vi "UHR-Fleezers Control (host) - Avogadro v2.vi"() -> ()   [LabVIEW 2014] (continued)
        n2315 = local read "Setpoints (V)"() -> (w3599:cluster{"Set 1":dbl, "Set 2":dbl})
        n2316 = Unbundle By Name(w3584) -> ("kappa_x (pN/nm)"=w3595:dbl, "kappa_y (pN/nm)"=w3594:dbl)
        n2317 = Unbundle By Name(w3591) -> ("kappa_x (pN/nm)"=w3593:dbl, "kappa_y (pN/nm)"=w3592:dbl)
        n2318 = Unbundle By Name(w3599) -> ("Set 1"=w3602:dbl, "Set 2"=w3601:dbl)
        n2319 = case shown="True" "Scale intensities" {
          tunnel: w3602 -> [w3616 w3629]
          tunnel: w3601 -> [w3615 w3622]
          tunnel: "Scaling factor" -> [w3612 w3617]
          tunnel: [w3614 w3628] -> w3597
          tunnel: [w3613 w3627] -> w3596
          tunnel: w3595 -> [w3611 w3623]
          tunnel: w3594 -> [w3610 w3624]
          tunnel: w3593 -> [w3609 w3625]
          tunnel: w3592 -> [w3608 w3626]
          tunnel: [w3607 w3621] -> w3590
          tunnel: [w3606 w3620] -> w3589
          tunnel: [w3605 w3619] -> w3588
          tunnel: [w3604 w3618] -> w3587
          frame False {
            n2320 = Divide(x=w3616, y=w3612) -> (x/y=w3614:dbl)
            n2321 = Divide(x=w3608, y=w3612) -> (x/y=w3604:dbl)
            n2322 = Divide(x=w3615, y=w3612) -> (x/y=w3613:dbl)
            n2323 = Divide(x=w3611, y=w3612) -> (x/y=w3607:dbl)
            n2324 = Divide(x=w3610, y=w3612) -> (x/y=w3606:dbl)
            n2325 = Divide(x=w3609, y=w3612) -> (x/y=w3605:dbl)
          }
          frame True {
            n2326 = Multiply(x=w3629, y=w3617) -> (x*y=w3628:dbl)
            n2327 = Multiply(x=w3622, y=w3617) -> (x*y=w3627:dbl)
            n2328 = Multiply(x=w3626, y=w3617) -> (x*y=w3618:dbl)
            n2329 = Multiply(x=w3623, y=w3617) -> (x*y=w3621:dbl)
            n2330 = Multiply(x=w3624, y=w3617) -> (x*y=w3620:dbl)
            n2331 = Multiply(x=w3625, y=w3617) -> (x*y=w3619:dbl)
          }
        }
        n2332 = Bundle By Name(cluster=w3584, "kappa_x (pN/nm)"=w3590, "kappa_y (pN/nm)"=w3589) -> (w3586:T12)
        n2333 = Bundle By Name(cluster=w3591, "kappa_x (pN/nm)"=w3588, "kappa_y (pN/nm)"=w3587) -> (w3585:T12)
        n2334 = Bundle By Name(cluster=w3599, "Set 1"=w3597, "Set 2"=w3596) -> (w3598:cluster{"Set 1":dbl, "Set 2":dbl})
        n2335 = property on="T1 calibration" class="Clust (strict)"("Val(Sgnl)"=w3586) -> ()  [unwired: 2 in, 2 out]
        n2336 = property on="T2 calibration" class="Clust (strict)"("Val(Sgnl)"=w3585) -> ()  [unwired: 2 in, 2 out]
        n2337 = property on="Setpoints (V)" class="Clust (strict)"("Val(Sgnl)"=w3598) -> ()  [unwired: 2 in, 2 out]
      }
      event "Piezo X at\n Scan position (V)": Value Change {
        n2338 = event-data() -> ()  [unwired: 7 out]
        n2339 = local read "AOM position for scan (MHz)"() -> (w3638:dbl)
        n2340 = local read "Piezo Trap X cal (nm/V)"() -> (w3632:dbl)
        n2341 = local read "AOM X Cal (nm/MHz)"() -> (w3635:dbl)
        n2342 = Subtract(x=w3638, y=60.0) -> (x-y=w3636:dbl)
        n2343 = Multiply(x=w3636, y=w3635) -> (x*y=w3633:dbl)
        n2344 = Multiply(x="Piezo X at\n Scan position (V)", y=w3632) -> (x*y=w3634:dbl)
        n2345 = Subtract(x=w3634, y=w3633) -> (x-y=w3631:dbl)
        n2346 = Divide(x=w3631, y=w3632) -> (x/y=→"Piezo trap x\noffset (V)":dbl)
      }
      event "Shift offset": Value Change {
        # "This events shifts the offset values by the currently measured values. For a quick way of correcting for changes in offsets"
        n2347 = event-data() -> ()  [unwired: 7 out]
        n2348 = local read "Multi-MCL offset array"() -> (w3661:T30)
        n2349 = local read "Offset file step size"() -> (w3649:dbl)
        n2350 = local read "MCL offset scanning range (V)"() -> (w3650:T4)
        n2351 = local write "Shift offset"(FALSE) -> ()
        n2352 = local read "Trap position array"() -> (w3662:dbl[])
        n2353 = Build Array(1, 0, 4, 3, 11, 10) -> (w3653:i32[])
        n2354 = local read "Values"() -> (w3654:dbl[])
        n2355 = for {
          tunnel: w3654 -> [w3666]
          tunnel: w3653 -> [w3665] mode=indexing
          tunnel: [w3664] -> w3652 mode=indexing
          n2356 = Index Array(array=w3666, index=w3665) -> (element=w3664:dbl)
        }
        n2357 = call "select offset array.vi"("MCL offset scanning range (V)"=w3650, "Offset File step size"=w3649, "Multi-MCL offset array"=w3661, "Trap position array"=w3662) -> ("Out offsets"=w3651:dbl[])  [unwired: 1 out]
        n2358 = Subtract(x=w3652, y=w3651) -> (x-y=w3641:dbl[])
        n2359 = local read "Raw offsets"() -> (w3648:dbl[])
        n2360 = Negate(x=w3641) -> (-x=w3640:dbl[])
        n2361 = call "generate multiple MCL offset.vi"("Offset array"=w3648, "offset file step size"=w3649, "MCL offset scanning range (V)"=w3650, "Corrections"=w3640) -> ("B_X mean out"=w3642:dbl[], "A_X mean out"=w3643:dbl[], "Output array"=w3647:T30)
        n2362 = local write "Multi-MCL offset array"(w3647) -> ()
        n2363 = local read "B factor"() -> (w3644:dbl)
        n2364 = Multiply(x=w3642, y=w3644) -> (x*y=w3646:dbl[])
        n2365 = Subtract(x=w3643, y=w3646) -> (x-y=w3645:dbl[])
        n2366 = property on="Setpoint offset\ncorrection values" class="Arr (strict)"("Val(Sgnl)"=w3645) -> ()  [unwired: 2 in, 2 out]
      }
    }
    "error out 2" <- w1816
    n2367 = node-c288() -> ()  [unwired: 2 out]
  }
  n2368 = node-c288() -> (w64:T42)  [unwired: 4 out]
  n2369 = timed-loop "Mouse control: trap position (AOM deflection), set confocal spot from image" {
    tunnel: [w3667] -> w69
    timing: w64 -> [_]
    timing-out: [_] -> w63
    tunnel: w26 -> [w3668]
    stop <- w3667 stop-if-true
    n2370 = node-c288() -> ()  [unwired: 2 out]
    n2371 = event shown="[0] \"Pane\": Mouse Down" {
      selector: _ -> [_ _ _ _]
      dyn-events: _ -> [_ _ _ _]
      timeout: _ -> [_ _ _ _]
      tunnel: w3668 -> [w3671 _ _ _]
      tunnel: [_ _ TRUE _] -> w3667
      event Mouse Down {
        n2372 = event-data() -> ("Time"=w3673:u32, "Coords"=w3672:T16, "Button"=w3674:u16)  [unwired: 6 out]
        n2373 = case shown="1" w3674 {
          tunnel: w3673 -> [_ _ w3799]
          tunnel: w3672 -> [_ w3711 w3797]
          tunnel: w3671 -> [_ _ w3793]
          frame 0, Default {
          }
          frame 1 {
            n2374 = property on="APD 2" class="ImageControl"() -> ("Displayed Image Position"=w3681:cluster{"Left":i32, "Top":i32})  [unwired: 2 in, 2 out]
            n2375 = property on="APD 1" class="ImageControl"() -> ("Displayed Image Position"=w3710:cluster{"Left":i32, "Top":i32})  [unwired: 2 in, 2 out]
            n2376 = property on="Detection Laser X" class="ImageControl"() -> ("Displayed Image Position"=w3707:cluster{"Left":i32, "Top":i32})  [unwired: 2 in, 2 out]
            n2377 = property on="Detection Laser Y" class="ImageControl"() -> ("Displayed Image Position"=w3706:cluster{"Left":i32, "Top":i32})  [unwired: 2 in, 2 out]
            n2378 = property on="APD 2" class="ImageControl"() -> ("Displayed Image Size"=w3680:cluster{"Width":u32, "Height":u32})  [unwired: 2 in, 2 out]
            n2379 = property on="APD 1" class="ImageControl"() -> ("Displayed Image Size"=w3708:cluster{"Width":u32, "Height":u32})  [unwired: 2 in, 2 out]
            n2380 = property on="Detection Laser X" class="ImageControl"() -> ("Displayed Image Size"=w3709:cluster{"Width":u32, "Height":u32})  [unwired: 2 in, 2 out]
            n2381 = property on="Detection Laser Y" class="ImageControl"() -> ("Displayed Image Size"=w3705:cluster{"Width":u32, "Height":u32})  [unwired: 2 in, 2 out]
            n2382 = Unbundle By Name(w3680) -> ("Width"=w3677:u32, "Height"=w3676:u32)
            n2383 = Unbundle By Name(w3681) -> ("Left"=w3679:i32, "Top"=w3678:i32)
            n2384 = Unbundle By Name(w3708) -> ("Width"=w3702:u32, "Height"=w3701:u32)
            n2385 = Unbundle By Name(w3709) -> ("Width"=w3698:u32, "Height"=w3697:u32)
            n2386 = Unbundle By Name(w3705) -> ("Width"=w3694:u32, "Height"=w3693:u32)
            n2387 = Unbundle By Name(w3710) -> ("Left"=w3704:i32, "Top"=w3703:i32)
            n2388 = Unbundle By Name(w3707) -> ("Left"=w3700:i32, "Top"=w3699:i32)
            n2389 = Unbundle By Name(w3706) -> ("Left"=w3696:i32, "Top"=w3695:i32)
            n2390 = Bundle("Left"=w3679, "Top"=w3678, "Width"=w3677, "Height"=w3676) -> (w3675:T58)  [unwired: 1 in]
            n2391 = Bundle("Left"=w3704, "Top"=w3703, "Width"=w3702, "Height"=w3701) -> (w3692:T58)  [unwired: 1 in]
            n2392 = Bundle("Left"=w3700, "Top"=w3699, "Width"=w3698, "Height"=w3697) -> (w3691:T58)  [unwired: 1 in]
            n2393 = Bundle("Left"=w3696, "Top"=w3695, "Width"=w3694, "Height"=w3693) -> (w3690:T58)  [unwired: 1 in]
            n2394 = Build Cluster Array(w3675, w3692, w3691, w3690) -> (w3689:T59)
            n2395 = for {
              tunnel: w3711 -> [w3722]
              tunnel: w3689 -> [w3723] mode=indexing
              shift-right: [w3720] -> w3687
              shift-left: TRUE -> [w3721]
              shift-right: [w3719] -> w3685
              shift-left: _ -> [w3715]
              shift-right: [w3718] -> w3684
              shift-left: _ -> [w3714]
              shift-right: [w3717] -> w3683
              shift-left: _ -> [w3713]
              shift-right: [w3716] -> w3682
              shift-left: _ -> [w3712]
              n2396 = case shown="True" w3721 {
                selector: w3721 -> [w3728 _]
                tunnel: w3723 -> [_ w3737]
                tunnel: w3722 -> [_ w3735]
                tunnel: [w3728 w3733] -> w3720
                tunnel: [w3727 w3732] -> w3719
                tunnel: [w3726 w3731] -> w3718
                tunnel: [w3725 w3730] -> w3717
                tunnel: [w3724 w3729] -> w3716
                tunnel: w3715 -> [w3727 _]
                tunnel: w3714 -> [w3726 _]
                tunnel: w3713 -> [w3725 _]
                tunnel: w3712 -> [w3724 _]
                frame False {
                }
                frame True {
                  n2397 = Unbundle(w3737) -> (w3736:T58)
                  n2398 = call "isclickinwindow.vi"("Image Param"=w3736, "Point32"=w3735) -> ("4 Y"=w3729:i32, "3 Height"=w3730:i32, "2 X"=w3731:i32, "1 Width"=w3732:i32, "In image?"=w3734:bool)  [unwired: 1 in]
                  n2399 = Not(x=w3734) -> (.not. x?=w3733:bool)
                }
              }
            }
            n2400 = Not(x=w3687) -> (.not. x?=w3686:bool)
            n2401 = case shown="True" w3686 {
              tunnel: w3684 -> [_ w3755]
              tunnel: w3682 -> [_ w3754]
              tunnel: w3685 -> [_ w3753]
              tunnel: w3683 -> [_ w3752]
              frame False {
              }
              frame True {
                w3742 = FALSE ("Get Point")
                n2402 = local read "Scan steps (MCL)"() -> (w3738:u64)
                n2403 = local read "Actual MCL Inc (V)"() -> (w3751:dbl)
                n2404 = local read "Scan lines (y)"() -> (w3756:u64)
                n2405 = Divide "Y Pix/step"(x=w3752, y=w3756) -> (x/y=w3762:dbl)
                n2406 = Divide "X pix/step"(x=w3753, y=w3738) -> (x/y=w3760:dbl)
                n2407 = Divide "Y V/pix"(x=w3751, y=w3762) -> (x/y=w3761:dbl)
                n2408 = local read "Initial Y"() -> (w3769:dbl)
                n2409 = Divide "Y half step offset"(x=w3751, y=2.0) -> (x/y=w3740:dbl)
                n2410 = Divide "X half step offset"(x=w3751, y=2.0) -> (x/y=w3758:dbl)
                n2411 = Divide "X V/pix"(x=w3751, y=w3760) -> (x/y=w3759:dbl)
                n2412 = Multiply(x=w3754, y=w3761) -> (x*y=w3770:dbl)
                n2413 = Negate(x=w3740) -> (-x=w3763:dbl)
                n2414 = Multiply(x=w3751, y=w3738) -> (x*y=w3765:dbl)
                n2415 = Multiply(x=w3759, y=w3755) -> (x*y=w3767:dbl)
                n2416 = Negate(x=w3758) -> (-x=w3757:dbl)
                n2417 = Compound Arithmetic op=ADD(w3763, w3770, w3769) -> (w3743:dbl)
                "Pointer Y (V)" <- w3743
                n2418 = local read "Initial X"() -> (w3768:dbl)
                n2419 = Negate(x=w3767) -> (-x=w3766:dbl)
                n2420 = Compound Arithmetic op=ADD(w3757, w3765, w3768, w3766) -> (w3744:dbl)
                "Pointer X (V)" <- w3744
                n2421 = case shown="True" "Set High F Confocal Spot (X-Y)" {
                  tunnel: w3744 -> [_ w3791]
                  tunnel: w3743 -> [_ w3792]
                  frame False {
                  }
                  frame True {
                    "Confocal Y 2 (V)" <- w3792
                    "Confocal X 2 (V)" <- w3791
                  }
                }
                n2422 = local read "Scan trap 3 or Fl?"() -> (w3741:bool)
                n2423 = Or(x="Set X Only", y="Set Confocal Spot (X-Y)") -> (x .or. y?=w3747:bool)
                n2424 = Or(x="Set Confocal Spot (X-Y)", y="Set Y Only") -> (x .or. y?=w3746:bool)
                n2425 = case shown="False" w3741 {
                  tunnel: w3747 -> [w3774 w3780]
                  tunnel: w3746 -> [w3773 w3779]
                  tunnel: w3744 -> [w3772 w3777]
                  tunnel: w3743 -> [w3771 w3778]
                  frame False {
                    n2426 = case shown="True" w3773 {
                      tunnel: w3771 -> [_ w3776]
                      frame False {
                      }
                      frame True {
                        n2427 = property on="AO1" class="Slide (strict)"("Val(Sgnl)"=w3776) -> ()  [unwired: 2 in, 2 out]
                        "Confocal Y 1 (V)" <- w3776
                      }
                    }
                    n2428 = case shown="True" w3774 {
                      tunnel: w3772 -> [_ w3775]
                      frame False {
                      }
                      frame True {
                        n2429 = property on="AO2" class="Slide (strict)"("Val(Sgnl)"=w3775) -> ()  [unwired: 2 in, 2 out]
                        "Confocal X 1 (V)" <- w3775
                      }
                    }
                  }
                  frame True {
                    n2430 = case shown="True" w3779 {
                      tunnel: w3778 -> [_ w3781]
                      frame False {
                      }
                      frame True {
                        n2431 = property on="Piezo trap y\noffset (V)" class="DigNum (strict)"("Val(Sgnl)"=w3781) -> ()  [unwired: 2 in, 2 out]
                      }
                    }
                    n2432 = case shown="True" w3780 {
                      tunnel: w3777 -> [_ w3786]
                      frame False {
                      }
                      frame True {
                        n2433 = local read "AOM X Cal (nm/MHz)"() -> (w3787:dbl)
                        n2434 = local read "Trap Delta (MHz)"() -> (w3789:dbl)
                        n2435 = Subtract(x=30.0, y=w3789) -> (x-y=w3788:dbl)
                        n2436 = Multiply(x=w3788, y=w3787) -> (x*y=w3784:dbl)
                        n2437 = local read "Piezo Trap X cal (nm/V)"() -> (w3783:dbl)
                        n2438 = Divide(x=w3784, y=w3783) -> (x/y=w3782:dbl)
                        n2439 = Subtract(x=w3786, y=w3782) -> (x-y=w3785:dbl)
                        n2440 = property on="Piezo trap x\noffset (V)" class="DigNum (strict)"("Val(Sgnl)"=w3785) -> ()  [unwired: 2 in, 2 out]
                      }
                    }
                  }
                }
                n2441 = local write "Set High F Confocal Spot (X-Y)"(w3742) -> ()
                n2442 = local write "Set Confocal Spot (X-Y)"(w3742) -> ()
                n2443 = local write "Set X Only"(w3742) -> ()
                n2444 = local write "Set Y Only"(w3742) -> ()
              }
            }
          }
          frame 3 {
            n2445 = local read "BD 2 Frequency 1 (MHz)"() -> (w3794:dbl)
            n2446 = local read "BD 1 Frequency 1 (MHz)"() -> (w3795:dbl)
            n2447 = local write "Manipulating Trap"(TRUE ("Manipulating Trap")) -> ()
            n2448 = local write "Coords"(T16 {"Horizontal"=0, "Vertical"=0} ("Coords")) -> ()
            n2449 = while {
              tunnel: w3799 -> [w3804]
              tunnel: w3797 -> [w3803]
              tunnel: w3795 -> [w3802]
              tunnel: w3794 -> [w3801]
              tunnel: w3793 -> [w3800]
              stop <- w3805 stop-if-true
              n2450 = event shown="[0] \"Pane\": Mouse Move" {
                selector: _ -> [_ _]
                dyn-events: _ -> [_ _]
                timeout: _ -> [_ _]
                tunnel: ["Force Manip Abort" w3869] -> w3805
                tunnel: w3804 -> [w3812 _]
                tunnel: w3803 -> [w3810 _]
                tunnel: w3802 -> [w3809 _]
                tunnel: w3801 -> [w3808 _]
                tunnel: w3800 -> [w3806 _]
                event Mouse Move {
                  n2451 = event-data() -> ("Time"=w3813:u32, "Coords"=w3814:T16)  [unwired: 3 out]
                  n2452 = Less?(x=w3813, y=w3812) -> (x < y?=w3811:bool)
                  n2453 = case "Makes sure old motion events prior to mouse click aren't used" shown="False" w3811 {
                    tunnel: w3814 -> [w3856 _]
                    tunnel: w3810 -> [w3857 _]
                    tunnel: w3809 -> [w3831 _]
                    tunnel: w3808 -> [w3830 _]
                    tunnel: w3806 -> [w3815 _]
                    frame False {
                      n2454 = Subtract(x=w3856, y=w3857) -> (x-y=w3855:T16)
                      "Coords" <- w3855
                      n2455 = local read "Y RF Frequency Limits (MHz)"() -> (w3816:T26)
                      n2456 = To Double Precision Float(number=w3855) -> (double precision float=w3854:cluster{"Horizontal":dbl, "Vertical":dbl})
                      n2457 = Multiply(x=cluster{"Horizontal":dbl, "Vertical":dbl} {"Horizontal"=-1.0, "Vertical"=1.0}, y="Manipulation Scaling") -> (x*y=w3850:cluster{"Horizontal":dbl, "Vertical":dbl})
                      n2458 = local read "X RF Frequency Limits (MHz)"() -> (w3817:T26)
                      n2459 = Multiply(x=w3854, y=w3850) -> (x*y=w3852:cluster{"Horizontal":dbl, "Vertical":dbl})
                      n2460 = Unbundle By Name(w3852) -> ("Horizontal"=w3847:dbl, "Vertical"=w3851:dbl)
                      n2461 = Unbundle By Name(w3816) -> ("Maximum"=w3819:dbl, "Minimum"=w3818:dbl)
                      n2462 = Boolean To (0,1)(Boolean="Manip. X?") -> (0, 1=w3845:i16)
                      n2463 = Boolean To (0,1)(Boolean="Manip. Y?") -> (0, 1=w3842:i16)
                      n2464 = local read "BD 1 Frequency 2 (MHz)"() -> (w3833:dbl)
                      n2465 = Multiply(x=w3851, y=w3842) -> (x*y=w3844:dbl)
                      n2466 = Multiply(x=w3845, y=w3847) -> (x*y=w3848:dbl)
                      n2467 = local read "BD 2 Frequency 2 (MHz)"() -> (w3832:dbl)
                      n2468 = Unbundle By Name(w3817) -> ("Maximum"=w3821:dbl, "Minimum"=w3820:dbl)
                      n2469 = Add(x=w3830, y=w3844) -> (x+y=w3823:dbl)
                      n2470 = Add(x=w3831, y=w3848) -> (x+y=w3825:dbl)
                      n2471 = In Range and Coerce(upper limit=w3821, x=w3825, lower limit=w3820) -> (coerced(x)=w3824:dbl)  [unwired: 1 out]
                      n2472 = In Range and Coerce(upper limit=w3819, x=w3823, lower limit=w3818) -> (coerced(x)=w3822:dbl)  [unwired: 1 out]
                      n2473 = Subtract(x=w3824, y=w3833) -> (x-y=w3841:dbl)
                      n2474 = Subtract(x=w3822, y=w3832) -> (x-y=w3840:dbl)
                      n2475 = Square(x=w3841) -> (x^2=w3839:dbl)
                      n2476 = Square(x=w3840) -> (x^2=w3838:dbl)
                      n2477 = Add(x=w3839, y=w3838) -> (x+y=w3837:dbl)
                      n2478 = Square Root(x=w3837) -> (sqrt(x)=w3834:dbl)
                      n2479 = In Range and Coerce(upper limit="Limit Max (MHz)", x=w3834, lower limit="Limit Min (MHz)") -> (In Range?=w3827:bool)  [unwired: 1 out]
                      n2480 = Not(x="Limits Enable") -> (.not. x?=w3826:bool)
                      n2481 = Or(x=w3827, y=w3826) -> (x .or. y?=w3828:bool)
                      n2482 = case shown="True" w3828 {
                        tunnel: w3834 -> [_ w3859]
                        tunnel: w3824 -> [_ w3866]
                        tunnel: w3833 -> [_ w3865]
                        tunnel: w3822 -> [_ w3864]
                        tunnel: w3832 -> [_ w3863]
                        tunnel: w3817 -> [_ w3861]
                        tunnel: w3816 -> [_ w3860]
                        tunnel: w3815 -> [_ w3858]
                        frame False {
                        }
                        frame True {
                          n2483 = local read "BD 1 Frequency 3 (MHz)"() -> (w3867:dbl)
                          n2484 = local read "BD 2 Frequency 3 (MHz)"() -> (w3862:dbl)
                          n2485 = local write "Trap Delta (MHz)"(w3859) -> ()
                          n2486 = call "set RF board frequency - interlace.vi"("Board 2 Frequency Limits"=w3860, "Board 1 Frequency Limits"=w3861, "FPGA VI Reference In"=w3858, "Board 2 Frequency 3 (MHz)"=w3862, "Board 1 Frequency 3 (MHz)"=w3867, "Board 2 Frequency 2 (MHz)"=w3863, "Board 2 Frequency 1 (MHz)"=w3864, "Board 1 Frequency 2 (MHz)"=w3865, "Board 1 Frequency 1  (MHz)"=w3866) -> ()  [unwired: 1 in, 2 out]
                          n2487 = local write "BD 2 Frequency 1 (MHz)"(w3864) -> ()
                          n2488 = local write "BD 1 Frequency 1 (MHz)"(w3866) -> ()
                        }
                      }
                    }
                    frame True {
                    }
                  }
                }
                event Mouse Up {
                  n2489 = event-data() -> ("Button"=w3868:u16)  [unwired: 8 out]
                  n2490 = case shown="3" w3868 {
                    tunnel: [FALSE TRUE] -> w3869
                    frame 0, Default {
                    }
                    frame 3 {
                      n2491 = local read "Trap Delta (MHz)"() -> (w3871:dbl)
                      n2492 = property on="Initial delta (MHz)" class="DigNum (strict)"("Val(Sgnl)"=w3871) -> ()  [unwired: 2 in, 2 out]
                      n2493 = local write "Manipulating Trap"(FALSE ("Manipulating Trap")) -> ()
                    }
                  }
                }
              }
            }
          }
        }
      }
      event Timeout {
        n2494 = event-data() -> ()  [unwired: 4 out]
      }
      event "Stop All": Mouse Down {
        n2495 = event-data() -> ()  [unwired: 9 out]
      }
      event Mouse Move {
        n2496 = event-data() -> ()  [unwired: 6 out]
      }
    }
    n2497 = node-c288() -> ()  [unwired: 2 out]
  }
  n2498 = node-c288(i64 1 ("Period"), 1 ("Processor")) -> (w68:T42)  [unwired: 2 in, 2 out]
  n2499 = node-c288(3 ("Processor")) -> (w60:T42)  [unwired: 3 out]
  n2500 = timed-loop "Oscillate Trap/AOM (fishing, conjugate plane alignment)" {
    tunnel: [w3877] -> w65
    timing: w60 -> [_]
    timing-out: [_] -> w59
    tunnel: w26 -> [w3876]
    tunnel: w3 -> [w3875]
    stop <- w3877 stop-if-true
    n2501 = node-c288() -> ()  [unwired: 2 out]
    n2502 = event shown="[2] \"Start assembly line\": Value Change" {
      selector: _ -> [_ _ _ _]
      dyn-events: _ -> [_ _ _ _]
      timeout: _ -> [_ _ _ _]
      tunnel: [FALSE ("Stop All") _ _ w4550] -> w3877
      tunnel: w3876 -> [w3880 _ _ _]
      tunnel: w3875 -> [_ _ w4485 _]
      event "Oscillate Set 1", "Fish for Tether": Value Change {
        n2503 = event-data() -> ()  [unwired: 6 out]
        n2504 = local read "Oscillate Set 1"() -> (w3884:bool)
        n2505 = Or(x=w3884, y="Fish for Tether") -> (x .or. y?=w3882:bool)
        n2506 = case shown="True" w3882 {
          tunnel: "Fish for Tether" -> [_ w3887]
          tunnel: w3880 -> [_ w3885]
          frame False {
          }
          frame True {
            n2507 = case shown="True" w3887 {
              selector: w3887 -> [w3890 w3896]
              tunnel: [w3890 w3896] -> w3886
              frame False {
              }
              frame True {
                n2508 = local write "Scan axis 2"(TRUE) -> ()
                n2509 = local write "Tether"(FALSE ("Tether")) -> ()
                n2510 = local read "Flow ON during cal?"() -> (w3891:bool)
                n2511 = property on="Trap Delta (MHz)" class="DigNum (strict)"("Val(Sgnl)"="Furthest Delta (MHz)") -> ()  [unwired: 2 in, 2 out]
                n2512 = Or(x="Flow ON during \nfishing?", y=w3891) -> (x .or. y?=w3892:bool)
                n2513 = Wait (ms)(milliseconds to wait=u32 500) -> ()  [unwired: 1 out]
                n2514 = property on="Sample Channel\nFlow" class="Bool (strict)"("Val(Sgnl)"=w3892) -> ()  [unwired: 2 in, 2 out]
              }
            }
            n2515 = node-c288() -> (w3889:T42)  [unwired: 1 in, 3 out]
            n2516 = timed-loop "Oscillate AOD" {
              timing: w3889 -> [_]
              timing-out: [_] -> w3888
              tunnel: w3886 -> [w3900]
              tunnel: w3885 -> [w3899]
              i -> [w3908]
              stop <- w3906 stop-if-true
              n2517 = node-c288() -> (w3907:i64)  [unwired: 1 out]
              n2518 = flat-sequence {
                tunnel: w3908 -> [w3935]
                tunnel: w3907 -> [w3934]
                tunnel: w3900 -> [w3918]
                tunnel: [w3918] -> w3905
                tunnel: [w3917] -> w3904
                tunnel: [w3916] -> w3903
                tunnel: [w3913] -> w3901
                tunnel: w3899 -> [w3909]
                tunnel: w3905 -> [w3982]
                tunnel: w3904 -> [w3980]
                tunnel: w3903 -> [w3979]
                tunnel: [w3978] -> w3902
                tunnel: w3901 -> [w3977]
                tunnel: [w4054] -> w3906
                tunnel: w3902 -> [w4053]
                frame #0 {
                  # "w (rad/s)"
                  # "t (s)"
                  n2519 = Divide(x=w3934, y=i64 1000) -> (x/y=w3910:dbl)
                  n2520 = local read "BD 1 Frequency 2 (MHz)"() -> (w3912:dbl)
                  n2521 = Multiply(x="Osc. freq. (Hz)", y=6.283185307179586) -> (x*y=w3932:dbl)
                  n2522 = Multiply(x=w3910, y=w3935) -> (x*y=w3931:dbl)
                  n2523 = Multiply(x=w3932, y=w3931) -> (x*y=w3915:dbl)
                  n2524 = local read "BD 1 Frequency 1 (MHz)"() -> (w3920:dbl)
                  n2525 = case shown="True" w3918 {
                    tunnel: w3915 -> [w3941 w3960]
                    tunnel: w3920 -> [_ w3968]
                    tunnel: w3912 -> [_ w3969]
                    tunnel: [w3938 w3964] -> w3911
                    tunnel: [FALSE w3942] -> w3916
                    tunnel: [0.0 w3956] -> w3913
                    frame False {
                      n2526 = Sine(x=w3941) -> (sin(x)=w3939:dbl)
                      n2527 = Multiply(x=w3939, y="Osc. amp. (MHz)") -> (x*y=w3938:dbl)
                    }
                    frame True {
                      # "trap position goes from 0 to 1 (0 is when it is furthest away, 1 is when closest)\nso we want to test for tether only when farther away, or x < 1"
                      # "quit if taking too long"
                      # "oscillate the trap"
                      # "Test for tether"
                      n2528 = local read "Vec Mean of T1 T2"() -> (w3945:dbl[])
                      "Trigger Signal" <- w3945
                      n2529 = Cosine(x=w3960) -> (cos(x)=w3972:dbl)
                      n2530 = Subtract(x=w3969, y=w3968) -> (x-y=w3967:dbl)
                      n2531 = Decrement(x=w3972) -> (x-1=w3971:dbl)
                      n2532 = Subtract(x=w3967, y="Closest Delta (MHz)") -> (x-y=w3965:dbl)
                      n2533 = Divide(x=w3971, y=-2.0) -> (x/y=w3955:dbl)
                      n2534 = Greater?(x=w3945, y="Stop F (pN)") -> (0:w3962:bool[])
                      n2535 = Multiply(x=w3955, y=w3965) -> (x*y=w3964:dbl)
                      n2536 = Less?(x=w3955, y="Fish mask thresh") -> (x < y?=w3954:bool)
                      n2537 = Boolean To (0,1)(Boolean=w3954) -> (0, 1=w3952:i16)
                      n2538 = Multiply(x=w3952, y=w3945) -> (x*y=w3951:dbl[])
                      n2539 = Divide(x=w3960, y=6.283185307179586) -> (x/y=w3959:dbl)
                      n2540 = Round Toward +Infinity(x=w3959) -> (ceil(x): smallest int >= x=w3956:dbl)
                      "Attempts" <- w3956
                      n2541 = Greater?(x=w3951, y="Stop F (pN) (mask)") -> (0:w3949:bool[])
                      n2542 = Or Array Elements(Boolean array=w3962) -> (logical OR=w3947:bool)
                      n2543 = Or Array Elements(Boolean array=w3949) -> (logical OR=w3946:bool)
                      n2544 = Greater?(x=w3956, y="Attempt Limit") -> (0:w3958:bool)
                      n2545 = case shown="True" w3958 {
                        frame False {
                        }
                        frame True {
                          n2546 = local write "Fish for Tether"(FALSE ("Fish for Tether")) -> ()
                          n2547 = call <vilib>:"Beep.vi"() -> ()  [unwired: 3 in, 9 out]
                          n2548 = local read "Messages"() -> (w3974:string)
                          n2549 = call "Update messages.vi"("Message to add"="Tether fishing timeout." ("Messages"), "Old message string"=w3974) -> ("New message string"=→"Messages":string)
                        }
                      }
                      n2550 = Select(t=w3947, s="Normal (on) or masked test (off)", f=w3946) -> (s? t:f=w3944:bool)
                      n2551 = And(x="Stop Fishing When Tether", y=w3944) -> (x .and. y?=w3942:bool)
                    }
                  }
                  n2552 = local read "BD 2 Frequency 1 (MHz)"() -> (w3919:dbl)
                  n2553 = Select(t=w3920, s="Scan axis 2", f=w3919) -> (s? t:f=w3923:dbl)
                  n2554 = Add(x=w3911, y=w3923) -> (x+y=w3917:dbl)
                  n2555 = Select(t=w3917, s="Scan axis 2", f=w3920) -> (s? t:f=w3926:dbl)
                  n2556 = Select(t=w3919, s="Scan axis 2", f=w3917) -> (s? t:f=w3925:dbl)
                  n2557 = local read "BD 2 Frequency 2 (MHz)"() -> (w3928:dbl)
                  n2558 = local read "BD 2 Frequency 3 (MHz)"() -> (w3927:dbl)
                  n2559 = local read "Y RF Frequency Limits (MHz)"() -> (w3921:T26)
                  n2560 = local read "X RF Frequency Limits (MHz)"() -> (w3922:T26)
                  n2561 = local read "BD 1 Frequency 3 (MHz)"() -> (w3929:dbl)
                  n2562 = call "set RF board frequency - interlace.vi"("Board 2 Frequency Limits"=w3921, "Board 1 Frequency Limits"=w3922, "FPGA VI Reference In"=w3909, "Board 2 Frequency 3 (MHz)"=w3927, "Board 1 Frequency 3 (MHz)"=w3929, "Board 2 Frequency 2 (MHz)"=w3928, "Board 2 Frequency 1 (MHz)"=w3925, "Board 1 Frequency 2 (MHz)"=w3912, "Board 1 Frequency 1  (MHz)"=w3926) -> ()  [unwired: 1 in, 2 out]
                }
                frame #1 {
                  n2563 = And(x=w3982, y=w3979) -> (x .and. y?=w3981:bool)
                  n2564 = case "Only if were fishing and now formed tether" shown="True" w3981 {
                    tunnel: w3980 -> [w3984 w3999]
                    tunnel: [w3983 w3998] -> w3978
                    tunnel: w3977 -> [_ w3994]
                    frame False {
                      n2565 = local read "Fish for Tether"() -> (w3983:bool)
                      n2566 = case shown="False" w3983 {
                        tunnel: w3984 -> [w3985 _]
                        frame False {
                          n2567 = property on="BD 1 Frequency 1 (MHz)" class="DigNum (strict)"("Val(Sgnl)"=w3985) -> ()  [unwired: 2 in, 2 out]
                        }
                        frame True {
                        }
                      }
                    }
                    frame True {
                      w3998 = FALSE ("Fish for Tether")
                      n2568 = call <vilib>:"Beep.vi"() -> ()  [unwired: 3 in, 9 out]
                      n2569 = Number To Decimal String(number=w3994, width (-)=i16 1) -> (decimal integer string=w3992:string)
                      n2570 = Concatenate Strings("Formed tether in ", w3992, " attempt(s)." ("string")) -> (w3989:string)
                      n2571 = local read "Messages"() -> (w3996:string)
                      n2572 = local write "Fish for Tether"(w3998) -> ()
                      n2573 = call "Update messages.vi"("Message to add"=w3989, "Old message string"=w3996) -> ("New message string"=w3995:string)
                      n2574 = local write "Messages"(w3995) -> ()
                      n2575 = Get Date/Time In Seconds() -> (seconds since 1Jan1904=→"Time tether formed":timestamp)
                      n2576 = local read "Flow ON during cal?"() -> (w3986:bool)
                      n2577 = property on="Sample Channel\nFlow" class="Bool (strict)"("Val(Sgnl)"=w3986) -> (error out=w3987:errorcluster)  [unwired: 2 in, 1 out]
                      n2578 = case shown="\"2\", \"3\", \"4\", \"5\", \"6\"" "Then..." {
                        selector: "Then..." -> [_ w4002]
                        tunnel: w3999 -> [w4001 _]
                        tunnel: w3987 -> [_ _]
                        frame "1", Default {
                          n2579 = property on="BD 1 Frequency 1 (MHz)" class="DigNum (strict)"("Val(Sgnl)"=w4001) -> ()  [unwired: 2 in, 2 out]
                        }
                        frame "2", "3", "4", "5", "6" {
                          n2580 = flat-sequence {
                            tunnel: w4002 -> [w4004]
                            frame #0 {
                              n2581 = property on="Trap Delta (MHz)" class="DigNum (strict)"("Val(Sgnl)"="Move to Delta 1 (MHz)") -> ()  [unwired: 2 in, 2 out]
                            }
                            frame #1 {
                              n2582 = case shown="\"5\", \"6\"" w4004 {
                                selector: w4004 -> [w4007 w4017 _]
                                frame "3", "4" {
                                n2583 = flat-sequence {
                                tunnel: w4007 -> [w4008]
                                tunnel: [w4008] -> w4005
                                tunnel: [w4010] -> w4006
                                tunnel: w4005 -> [w4010]
                                tunnel: w4006 -> [w4014]
                                frame #0 {
                                n2584 = property on="Green Laser ON" class="Bool (strict)"("Val(Sgnl)"=TRUE ("Value (Signaling)")) -> ()  [unwired: 2 in, 2 out]
                                }
                                frame #1 {
                                n2585 = Multiply(x="Wait Before Save (s)", y=u32 1000 ("x")) -> (x*y=w4012:u32)
                                n2586 = Wait (ms)(milliseconds to wait=w4012) -> ()  [unwired: 1 out]
                                }
                                frame #2 {
                                n2587 = property on="Start Saving" class="Bool (strict)"("Value"=TRUE ("Start Saving")) -> ()  [unwired: 2 in, 2 out]
                                n2588 = case shown="\"4\"" w4014 {
                                frame Default {
                                }
                                frame "4" {
                                n2589 = property on="Fl. Triggered..." class="Bool (strict)"("Val(Sgnl)"=TRUE ("Value (Signaling)")) -> ()  [unwired: 2 in, 2 out]
                                }
                                }
                                }
                                }
                                }
                                frame "5", "6" {
                                n2590 = stacked-sequence {
                                tunnel: w4017 -> [_ _ _ _ _ _ w4029]
                                frame #0 {
                                n2591 = Replace Array Subset(array=u32[] [0] ("Index Values"), new element="Raster Set Upon Tether", index=0) -> (w4018:u32[])
                                n2592 = property on="Saved AOD Raster Scan Parameter Sets" class="Arr (strict)"("Index Values"=w4018) -> ()  [unwired: 2 in, 2 out]
                                }
                                frame #1 {
                                n2593 = Wait (ms)(milliseconds to wait=u32 500) -> ()  [unwired: 1 out]
                                }
                                frame #2 {
                                n2594 = property on="Load parameters" class="Bool (strict)"("Val(Sgnl)"=TRUE ("Value (Signaling)")) -> ()  [unwired: 2 in, 2 out]
                                n2595 = case shown="True" "Green ON During Raster" {
                                frame False {
                                }
                                frame True {
                                n2596 = property on="Green Laser ON" class="Bool (strict)"("Val(Sgnl)"=TRUE ("Value (Signaling)")) -> ()  [unwired: 2 in, 2 out]
                                }
                                }
                                }
                                frame #3 {
                                n2597 = Wait (ms)(milliseconds to wait=u32 500) -> ()  [unwired: 1 out]
                                }
                                frame #4 {
                                n2598 = property on="Trap Raster Scan" class="Bool (strict)"("Val(Sgnl)"=TRUE ("Value (Signaling)")) -> ()  [unwired: 2 in, 2 out]
                                }
                                frame #5 {
                                n2599 = Wait (ms)(milliseconds to wait=u32 2000) -> ()  [unwired: 1 out]
                                }
                                frame #6 {
                                n2600 = flat-sequence {
                                tunnel: w4029 -> [w4036]
                                frame #0 {
                                n2601 = while {
                                stop <- w4032 stop-if-true
                                n2602 = local read "Raster Scanning..."() -> (w4031:bool)
                                n2603 = local read "Saving..."() -> (w4034:bool)
                                n2604 = Wait (ms)(milliseconds to wait=u32 100) -> ()  [unwired: 1 out]
                                n2605 = Not(x=w4034) -> (.not. x?=w4033:bool)
                                n2606 = Not(x=w4031) -> (.not. x?=w4030:bool)
                                n2607 = And(x=w4033, y=w4030) -> (x .and. y?=w4032:bool)
                                }
                                }
                                frame #1 {
                                n2608 = local read "Tether"() -> (w4037:bool)
                                n2609 = case shown="True" w4037 {
                                tunnel: w4036 -> [_ w4039]
                                frame False {
                                n2610 = property on="Fish for Tether" class="Bool (strict)"("Val(Sgnl)"="Fish again after \nraster break?") -> ()  [unwired: 2 in, 2 out]
                                }
                                frame True {
                                n2611 = stacked-sequence {
                                tunnel: w4039 -> [_ w4043 _ _]
                                frame #0 {
                                n2612 = property on="Trap Delta (MHz)" class="DigNum (strict)"("Val(Sgnl)"="Move to Delta 2 (MHz)") -> ()  [unwired: 2 in, 2 out]
                                n2613 = case shown="True" "Flow ON after\ntether testing?" {
                                frame False {
                                }
                                frame True {
                                n2614 = property on="Sample Channel\nFlow" class="Bool (strict)"("Val(Sgnl)"=TRUE ("Value (Signaling)")) -> ()  [unwired: 2 in, 2 out]
                                }
                                }
                                }
                                frame #1 {
                                n2615 = flat-sequence {
                                tunnel: w4043 -> [w4045]
                                frame #0 {
                                n2616 = Wait (ms)(milliseconds to wait=u32 500) -> ()  [unwired: 1 out]
                                }
                                frame #1 {
                                n2617 = case shown="\"6\"" w4045 {
                                frame Default {
                                }
                                frame "6" {
                                n2618 = property on="Green Laser ON" class="Bool (strict)"("Val(Sgnl)"=TRUE ("Green Laser ON/Interlacing")) -> ()  [unwired: 2 in, 2 out]
                                }
                                }
                                }
                                frame #2 {
                                n2619 = Wait (ms)(milliseconds to wait=u32 500) -> ()  [unwired: 1 out]
                                }
                                frame #3 {
                                n2620 = local write "Start Saving"("Save at end (5, 6)") -> ()
                                }
                                }
                                }
                                frame #2 {
                                n2621 = local read "Bead Sep. Int. Time (s)"() -> (w4051:dbl)
                                n2622 = Multiply(x=w4051, y=1000.0) -> (x*y=w4050:dbl)
                                n2623 = Wait (ms)(milliseconds to wait=w4050) -> ()  [unwired: 1 out]
                                }
                                frame #3 {
                                n2624 = property on="Remove Offset" class="Bool (strict)"("Val(Sgnl)"=TRUE ("Value (Signaling)")) -> ()  [unwired: 2 in, 2 out]
                                }
                                }
                                }
                                }
                                }
                                }
                                }
                                }
                                }
                                frame "2", Default {
                                }
                              }
                            }
                          }
                        }
                      }
                      "Tether" <- "Tether Alarm?"
                    }
                  }
                }
                frame #2 {
                  n2625 = local read "Oscillate Set 1"() -> (w4058:bool)
                  n2626 = local read "Stop All"() -> (w4056:bool)
                  n2627 = Or(x=w4058, y=w4053) -> (x .or. y?=w4055:bool)
                  n2628 = Not(x=w4055) -> (.not. x?=w4057:bool)
                  n2629 = Compound Arithmetic op=OR(w4056, w4057) -> (w4054:bool)
                }
              }
              n2630 = node-c288() -> ()  [unwired: 2 out]
            }
            n2631 = node-c288(w3888) -> ()  [unwired: 1 out]
          }
        }
      }
      event "Fl. Triggered...": Value Change {
        n2632 = event-data() -> ()  [unwired: 7 out]
        n2633 = case shown="True" "Fl. Triggered..." {
          frame False {
          }
          frame True {
            n2634 = node-c288() -> (w4069:T42)  [unwired: 4 out]
            n2635 = timed-loop {
              timing: w4069 -> [_]
              timing-out: [_] -> w4068
              tunnel: "Action" -> [w4077]
              shift-right: [w4074] -> _
              shift-left: u8 255 -> [w4076]
              shift-right: [w4071] -> _
              shift-left: 255 -> [w4073]
              stop <- w4070 stop-if-true
              # "Reset confocal spot"
              n2636 = node-c288() -> ()  [unwired: 2 out]
              n2637 = flat-sequence {
                tunnel: w4077 -> [w4097]
                tunnel: w4076 -> [w4096]
                tunnel: [w4095] -> w4075
                tunnel: w4073 -> [w4082]
                tunnel: [w4081] -> w4072
                tunnel: [w4476] -> w4070
                tunnel: w4075 -> [w4475]
                tunnel: [w4475] -> w4074
                tunnel: [w4474] -> w4071
                tunnel: w4072 -> [w4474]
                frame #0 {
                  n2638 = local read "Delta Fl. 2"() -> (w4094:dbl)
                  n2639 = local read "Delta Fl. 1"() -> (w4089:dbl)
                  n2640 = Multiply(x="Fl. Delta Thresh. (kHz)", y=1000.0) -> (x*y=w4084:dbl)
                  n2641 = Select(t=w4089, s="APD to Watch", f=w4094) -> (s? t:f=w4085:dbl)
                  n2642 = Greater?(x=w4085, y=w4084) -> (0:w4090:bool)
                  n2643 = Or(x="Force Yank", y=w4090) -> (x .or. y?=w4088:bool)
                  n2644 = And(x=w4088, y="Yank when?") -> (x .and. y?=w4086:bool)
                  n2645 = case shown="False" w4086 {
                    tunnel: w4097 -> [w4100 w4301]
                    tunnel: w4096 -> [w4102 w4297]
                    tunnel: [w4102 w4295] -> w4095
                    tunnel: w4085 -> [w4108 _]
                    tunnel: w4084 -> [w4107 _]
                    tunnel: "Force Yank" -> [w4105 _]
                    tunnel: w4082 -> [w4104 w4294]
                    tunnel: [w4103 w4294] -> w4081
                    frame False {
                      n2646 = Negate(x=w4107) -> (-x=w4099:dbl)
                      n2647 = local write "Fl. High"(TRUE ("Fl. High")) -> ()
                      n2648 = Less?(x=w4108, y=w4099) -> (x < y?=w4106:bool)
                      n2649 = Or(x=w4105, y=w4106) -> (x .or. y?=w4101:bool)
                      n2650 = case shown="True" w4101 {
                        tunnel: w4104 -> [w4109 w4119]
                        tunnel: [w4109 w4118] -> w4103
                        tunnel: w4100 -> [_ w4117]
                        frame False {
                        }
                        frame True {
                          n2651 = flat-sequence {
                            tunnel: w4119 -> [w4125]
                            tunnel: w4117 -> [w4122]
                            tunnel: [w4124] -> w4116
                            tunnel: [w4123] -> w4115
                            tunnel: [w4122] -> w4114
                            tunnel: w4113 -> [w4121]
                            tunnel: [w4121] -> w4112
                            tunnel: w4111 -> [w4120]
                            tunnel: [w4120] -> w4110
                            tunnel: [w4196] -> w4118
                            tunnel: w4116 -> [w4196]
                            tunnel: w4115 -> [w4195]
                            tunnel: w4114 -> [w4194]
                            tunnel: w4112 -> [w4193]
                            tunnel: w4110 -> [w4192]
                            frame #0 {
                              n2652 = call <vilib>:"Beep.vi"() -> ()  [unwired: 12 in]
                              n2653 = local write "Waiting"(FALSE ("Waiting")) -> ()
                              n2654 = Increment(x=w4125) -> (x+1=w4124:i32)
                              n2655 = case shown="\"Yank\"" w4122 {
                                tunnel: w4124 -> [_ w4130 _]
                                frame "Alarm", Default {
                                }
                                frame "Yank" {
                                n2656 = flat-sequence {
                                tunnel: w4130 -> [w4133]
                                tunnel: [w4132] -> w4129
                                tunnel: [w4131] -> w4128
                                tunnel: w4129 -> [w4143]
                                tunnel: w4128 -> [w4144]
                                frame #0 {
                                n2657 = local read "Yank Delay (s)"() -> (w4136:dbl)
                                n2658 = local read "N Array El"() -> (w4131:u8)
                                n2659 = Quotient & Remainder(x=w4133, y=w4131) -> (x-y*floor(x/y)=w4132:i32)  [unwired: 1 out]
                                n2660 = Multiply(x=w4136, y=1000.0) -> (x*y=w4134:dbl)
                                n2661 = Wait (ms)(milliseconds to wait=w4134) -> ()  [unwired: 1 out]
                                }
                                frame #1 {
                                n2662 = local read "Yank to which?"() -> (w4138:bool)
                                n2663 = local read "Random Choice"() -> (w4148:bool)
                                n2664 = local read "Yank to Trap Delta (MHz)"() -> (w4141:dbl[])
                                n2665 = local read "Yank to SP"() -> (w4142:dbl[])
                                n2666 = Random Number (0-1)() -> (number: 0 to 1=w4147:dbl)
                                n2667 = Multiply(x=w4144, y=w4147) -> (x*y=w4146:dbl)
                                n2668 = Round Toward -Infinity(1:w4146) -> (0:w4145:dbl)
                                n2669 = Select(t=w4145, s=w4148, f=w4143) -> (s? t:f=w4139:dbl)
                                n2670 = Select(t=w4141, s=w4138, f=w4142) -> (s? t:f=w4140:dbl[])
                                n2671 = Index Array(array=w4140, index=w4139) -> (element=w4137:dbl)
                                n2672 = case shown="False" w4138 {
                                tunnel: w4137 -> [w4149 w4176]
                                frame False {
                                n2673 = flat-sequence {
                                tunnel: w4149 -> [w4150]
                                frame #0 {
                                n2674 = property on="Trap Pos FB SP" class="DigNum (strict)"("Val(Sgnl)"=w4150) -> ()  [unwired: 2 in, 2 out]
                                }
                                frame #1 {
                                n2675 = Wait (ms)(milliseconds to wait=u32 700) -> ()  [unwired: 1 out]
                                }
                                frame #2 {
                                n2676 = local read "Action (%)"() -> (w4155:dbl)
                                n2677 = Absolute Value(x=w4155) -> (abs(x)=w4154:dbl)
                                n2678 = Greater?(x=w4154, y=70.0) -> (0:w4152:bool)
                                n2679 = property on="Remove Action Offset" class="Bool (strict)"("Val(Sgnl)"=w4152) -> ()  [unwired: 2 in, 2 out]
                                }
                                frame #3 {
                                n2680 = for {
                                N: 4 -> [_]
                                n2681 = flat-sequence {
                                frame #0 {
                                n2682 = Wait (ms)(milliseconds to wait=u32 500) -> ()  [unwired: 1 out]
                                }
                                frame #1 {
                                n2683 = local read "Action (%)"() -> (w4161:dbl)
                                n2684 = Absolute Value(x=w4161) -> (abs(x)=w4160:dbl)
                                n2685 = Greater?(x=w4160, y=70.0) -> (0:w4158:bool)
                                n2686 = property on="Remove Action Offset" class="Bool (strict)"("Val(Sgnl)"=w4158) -> ()  [unwired: 2 in, 2 out]
                                }
                                }
                                }
                                }
                                frame #4 {
                                n2687 = Wait (ms)(milliseconds to wait=u32 500) -> ()  [unwired: 1 out]
                                }
                                frame #5 {
                                n2688 = local read "Mean"() -> (w4169:dbl)
                                n2689 = Greater?(x=w4169, y=11.0) -> (0:w4163:bool)
                                n2690 = Not(x=w4163) -> (.not. x?=w4164:bool)
                                n2691 = And(x=w4164, y="Shift confocal") -> (x .and. y?=w4166:bool)
                                n2692 = And(x=w4163, y="Shift confocal") -> (x .and. y?=w4167:bool)
                                n2693 = case shown="True" w4167 {
                                frame False {
                                }
                                frame True {
                                n2694 = local read "Confocal Y 2 (V)"() -> (w4173:dbl)
                                n2695 = local read "Confocal X 2 (V)"() -> (w4172:dbl)
                                n2696 = property on="AO1" class="Slide (strict)"("Val(Sgnl)"=w4173) -> ()  [unwired: 2 in, 2 out]
                                n2697 = property on="AO2" class="Slide (strict)"("Val(Sgnl)"=w4172) -> ()  [unwired: 2 in, 2 out]
                                }
                                }
                                n2698 = case shown="True" w4166 {
                                frame False {
                                }
                                frame True {
                                n2699 = local read "Confocal Y 1 (V)"() -> (w4171:dbl)
                                n2700 = local read "Confocal X 1 (V)"() -> (w4170:dbl)
                                n2701 = property on="AO1" class="Slide (strict)"("Val(Sgnl)"=w4171) -> ()  [unwired: 2 in, 2 out]
                                n2702 = property on="AO2" class="Slide (strict)"("Val(Sgnl)"=w4170) -> ()  [unwired: 2 in, 2 out]
                                }
                                }
                                }
                                frame #6 {
                                n2703 = Wait (ms)(milliseconds to wait=u32 1500) -> ()  [unwired: 1 out]
                                }
                                frame #7 {
                                n2704 = property on="Rem fb disp offset" class="Bool (strict)"("Val(Sgnl)"=TRUE ("Value (Signaling)")) -> ()  [unwired: 2 in, 2 out]
                                }
                                }
                                }
                                frame True {
                                n2705 = flat-sequence {
                                tunnel: w4176 -> [w4177]
                                frame #0 {
                                n2706 = property on="Trap Delta (MHz)" class="DigNum (strict)"("Val(Sgnl)"=w4177) -> ()  [unwired: 2 in, 2 out]
                                }
                                frame #1 {
                                n2707 = Wait (ms)(milliseconds to wait=u32 500) -> ()  [unwired: 1 out]
                                }
                                frame #2 {
                                n2708 = local read "Shift confocal"() -> (w4183:bool)
                                n2709 = local read "Mean"() -> (w4185:dbl)
                                n2710 = Greater?(x=w4185, y=11.0) -> (0:w4182:bool)
                                n2711 = Not(x=w4182) -> (.not. x?=w4181:bool)
                                n2712 = And(x=w4181, y=w4183) -> (x .and. y?=w4179:bool)
                                n2713 = And(x=w4182, y=w4183) -> (x .and. y?=w4180:bool)
                                n2714 = case shown="True" w4180 {
                                frame False {
                                }
                                frame True {
                                n2715 = local read "Confocal Y 2 (V)"() -> (w4189:dbl)
                                n2716 = local read "Confocal X 2 (V)"() -> (w4188:dbl)
                                n2717 = property on="AO2" class="Slide (strict)"("Val(Sgnl)"=w4188) -> ()  [unwired: 2 in, 2 out]
                                n2718 = property on="AO1" class="Slide (strict)"("Val(Sgnl)"=w4189) -> ()  [unwired: 2 in, 2 out]
                                }
                                }
                                n2719 = case shown="True" w4179 {
                                frame False {
                                }
                                frame True {
                                n2720 = local read "Confocal X 1 (V)"() -> (w4186:dbl)